vi "CRYO_MASTER_temp.vi"() -> ()   [LabVIEW 2017] (continued)
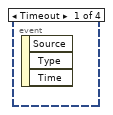
[diagram p2: hidden frame]
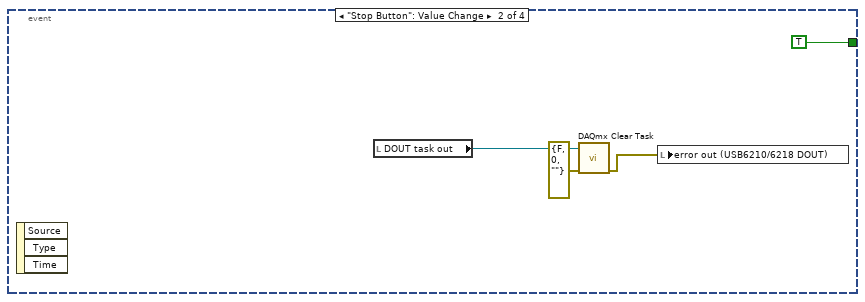
[diagram p3: hidden frame]
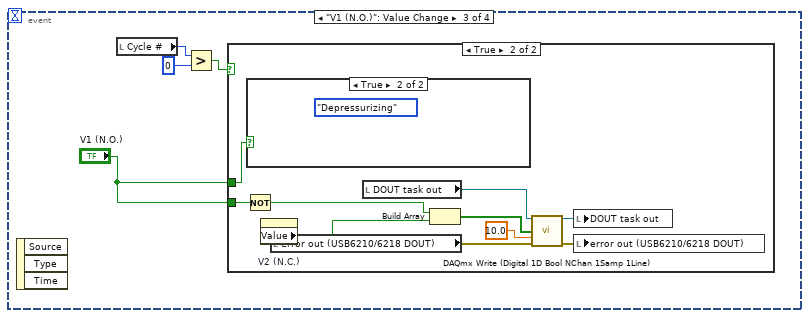
[diagram p4: hidden frame]
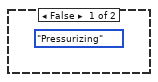
[diagram p6: hidden frame]
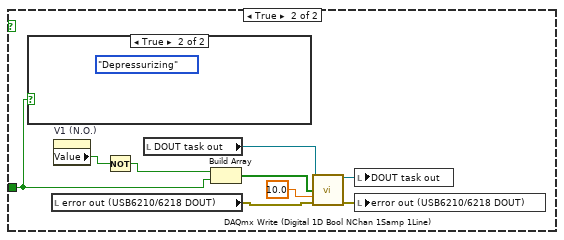
[diagram p7: hidden frame]
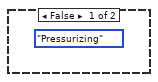
[diagram p8: hidden frame]
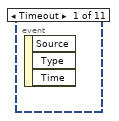
[diagram p9: hidden frame]
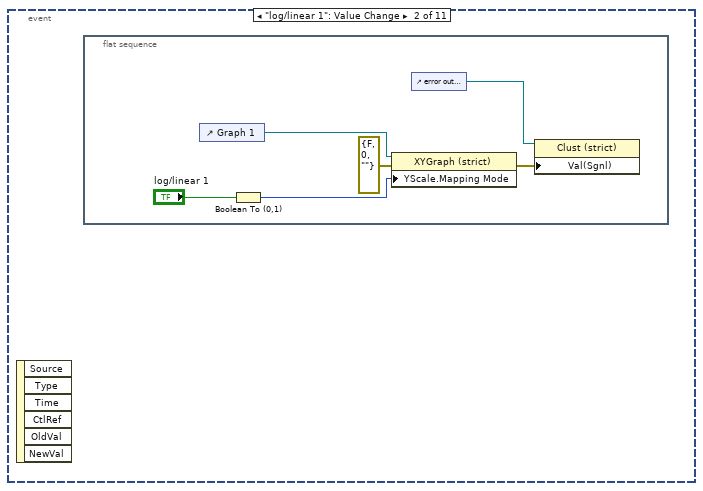
[diagram p10: hidden frame]
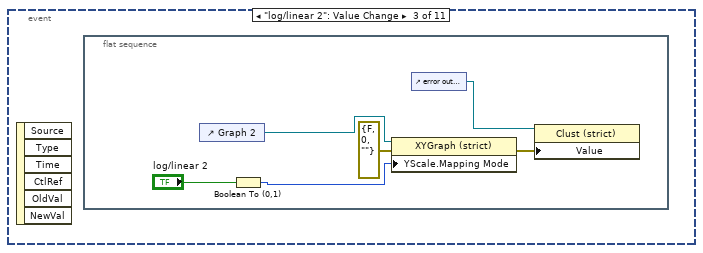
[diagram p11: hidden frame]
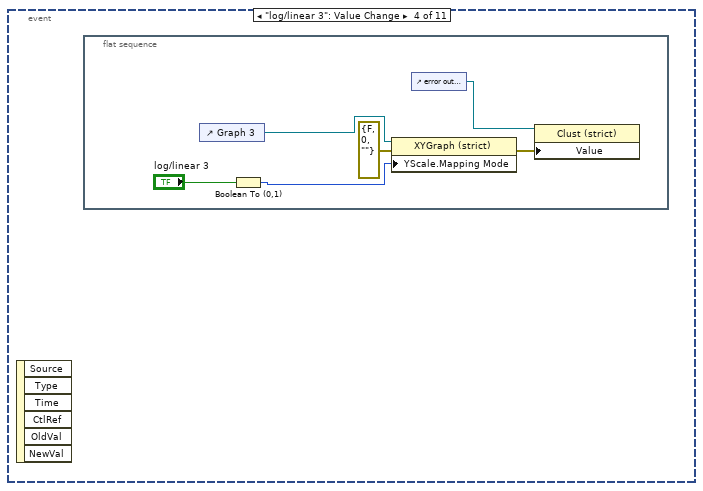
[diagram p12: hidden frame]
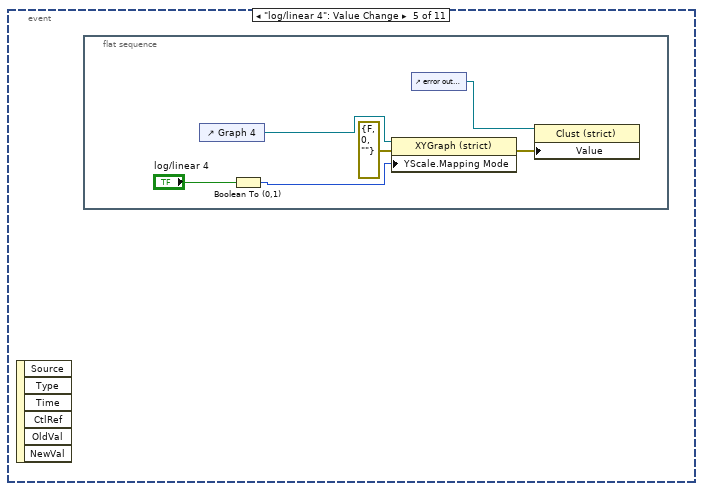
[diagram p13: hidden frame]
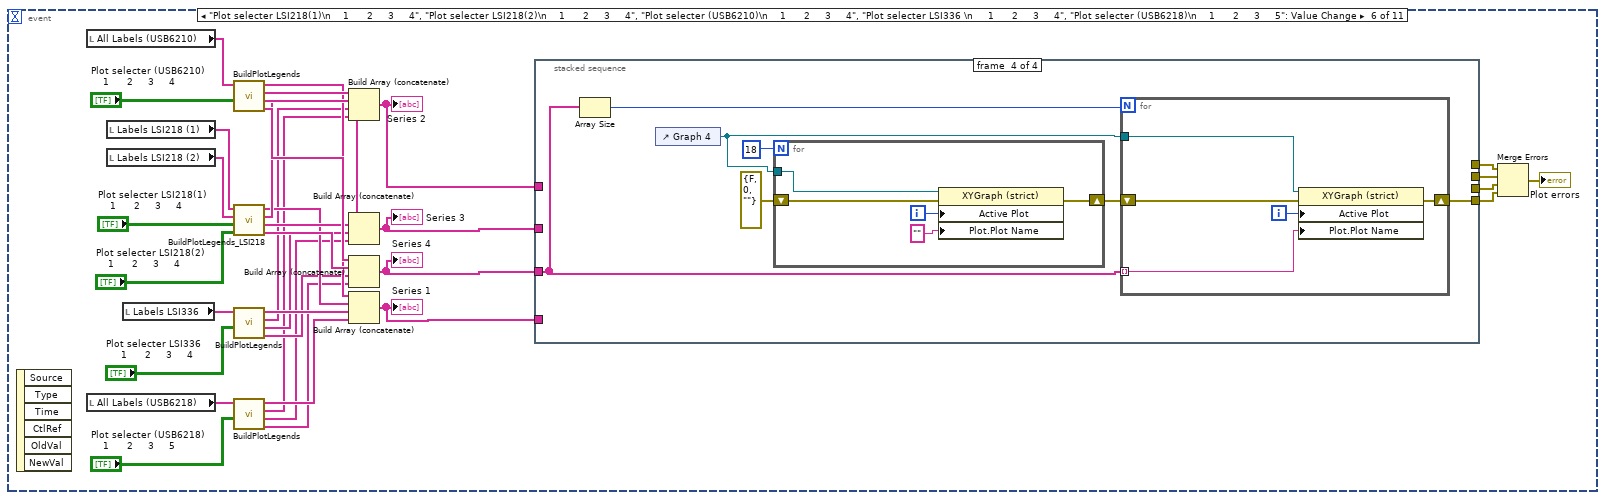
[diagram p14: hidden frame]
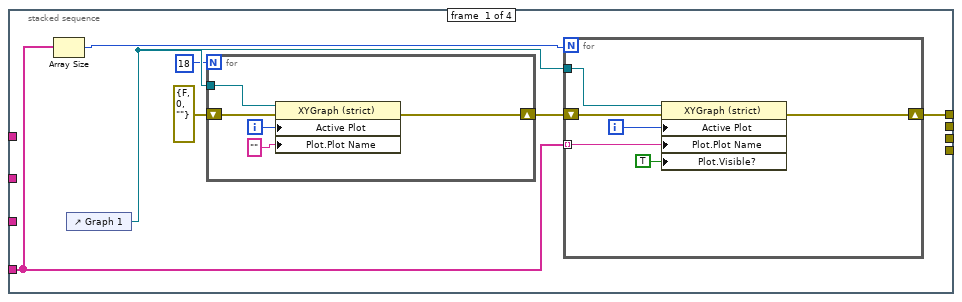
[diagram p15: hidden frame]
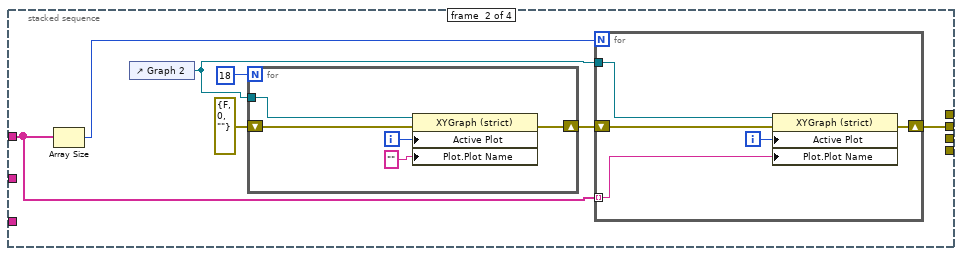
[diagram p16: hidden frame]
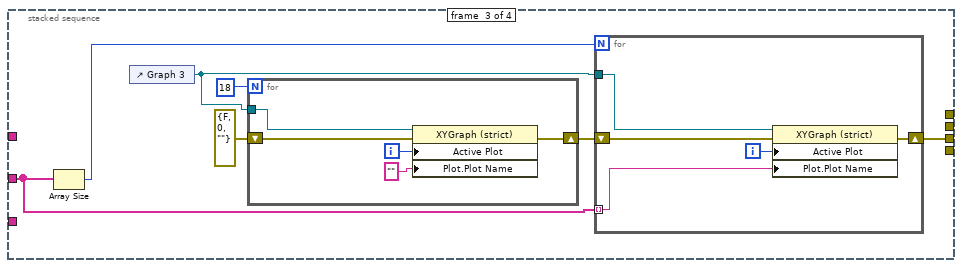
[diagram p17: hidden frame]
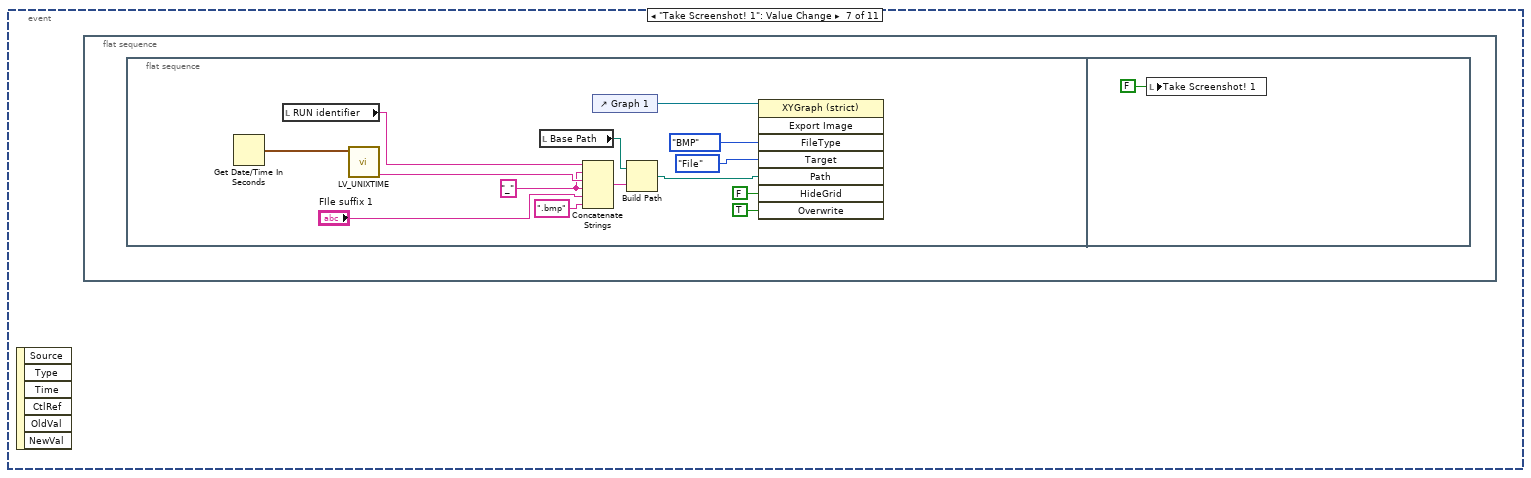
[diagram p18: hidden frame]
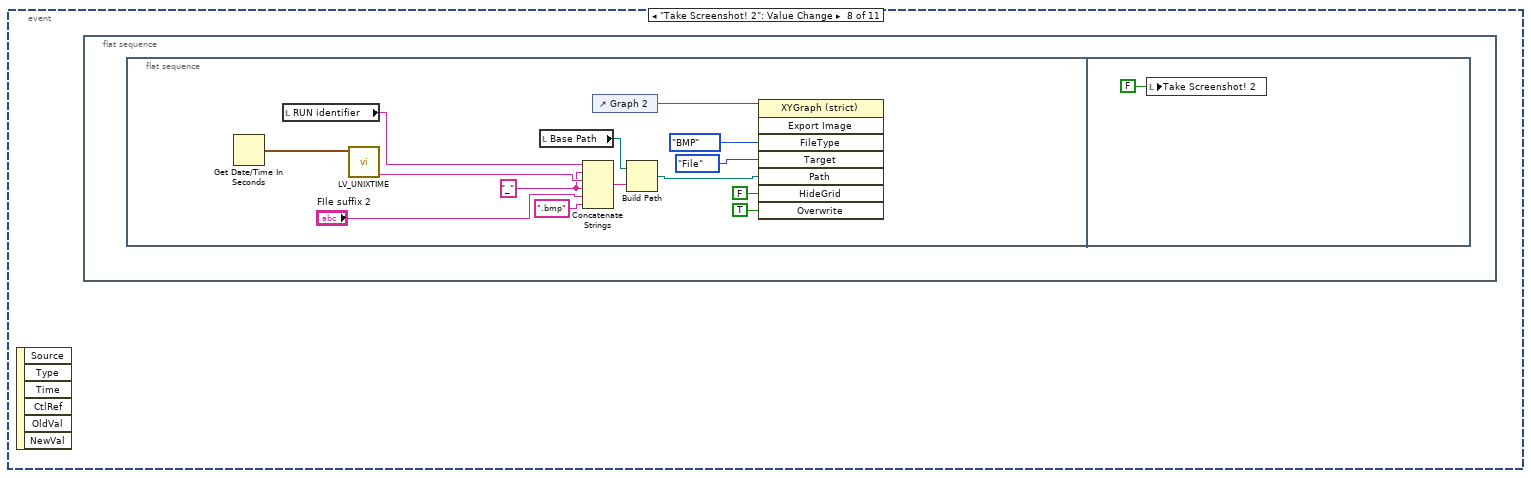
[diagram p19: hidden frame]
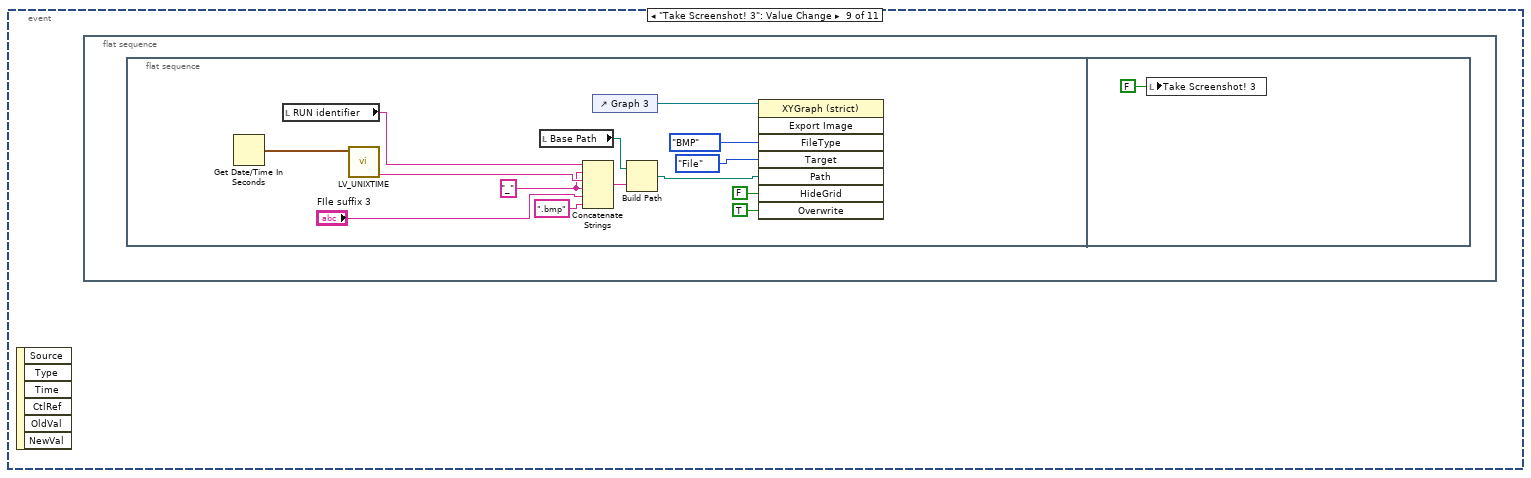
[diagram p20: hidden frame]
      }
    }
    "LSI336 Status" <- w289
    "error out (LSI336)" <- w279
    n190 = case shown="False" w264 {
      tunnel: [w502 w530] -> w252
      tunnel: [w499 w529] -> w259
      tunnel: [w500 w528] -> w253
      tunnel: [w490 w523] -> w258
      tunnel: [w489 w520] -> _
      tunnel: w265 -> [w488 w518]
      tunnel: w263 -> [_ w517]
      tunnel: w262 -> [_ w516]
      tunnel: w261 -> [w487 w515]
      tunnel: w260 -> [w486 _]
      frame False {
        n191 = call-dynamic "USBData_measure.vi"("USBData in"=w488, "DAQ sample #"=i64 5, "DAQ timeout"=100.0 ("DAQ timeout (def: 100)"), "MeasurementIndex"=w486, "error in (no error)"=w487) -> ("USBData out"=w508:refnum<class "USBData.lvclass">, "TimeMeasuremeent"=w505:timestamp, "Status"=→"USB6218 Status":T5, "LastDataAcquired"=w492:dbl[], "error out"=w504:errorcluster)  [unwired: 4 in, 2 out]
        "Time of Last Measurement (USB6218)" <- w505
        "Last Vol \n(USB6218)" <- w492
        n192 = call-dynamic "USBData_convert.vi"("Save every ... measurements"="Record interval (USB6218)", "MeasurementIndex"=w486, "error in (no error)"=w504, "LastDataAcquired"=w492, "TimeMeasuremeent"=w505, "USBData in"=w508) -> ("error out"=w503:errorcluster, "LeakDet_FULL"=w498:dbl, "LastDataConverted"=w493:dbl[], "USBData out"=w501:refnum<class "USBData.lvclass">)  [unwired: 2 in]
        n193 = call "USBData_read.vi"("USBData in"=w501, "error in (no error)"=w503) -> ("Status"=w494:T5, "USBData out"=w500:refnum<class "USBData.lvclass">, "Data"=w499:T13, "Basic"=w490:T14, "error out"=w502:errorcluster)  [unwired: 2 in, 2 out]
        n194 = local write "USB6218 Status"(w494) -> ()
        n195 = Unbundle By Name(w490) -> ("ReadLeakDet?"=w497:bool)
        n196 = Unbundle By Name(w490) -> ("Labels"=w489:string[])
        n197 = case shown="True" w497 {
          tunnel: w493 -> [w509 w512]
          tunnel: w498 -> [_ w511]
          tunnel: [w509 w510] -> w496
          frame False {
          }
          frame True {
            n198 = Build Array (concatenate)(w512, w511) -> (w510:dbl[])
          }
        }
        "Last Data \n(USB6218)" <- w496
      }
      frame True {
        n199 = Get Date/Time In Seconds() -> (seconds since 1Jan1904=w522:timestamp)
        n200 = call-dynamic "USBData_initialize.vi"("USBData in"=w518, "SeriesSetting"="USB6218 Config", "BasePath"=w517, "RunName"=w516, "FileName"="InstName (USB6218)", "error in (no error)"=w515, "RUN start time"=w522) -> ("Status"=w513:T5, "USBData out"=w531:refnum<class "USBData.lvclass">, "error out"=w532:errorcluster)  [unwired: 4 in, 2 out]
        n201 = local write "USB6218 Status"(w513) -> ()
        n202 = call "USBData_read.vi"("USBData in"=w531, "error in (no error)"=w532) -> ("Status"=w521:T5, "USBData out"=w528:refnum<class "USBData.lvclass">, "Data"=w529:T13, "Basic"=w523:T14, "error out"=w530:errorcluster)  [unwired: 2 in, 2 out]
        n203 = local write "USB6218 Status"(w521) -> ()
        n204 = Unbundle By Name(w523) -> ("ReadLeakDet?"=w527:bool, "Labels"=w520:string[])
        n205 = Array Size(array=w520) -> (size(s)=w526:i32)
        n206 = case shown="True" w527 {
          tunnel: w526 -> [w533 w535]
          tunnel: [w533 w534] -> w524
          frame False {
          }
          frame True {
            n207 = Add(x=w535, y=1) -> (x+y=w534:i32)
          }
        }
        n208 = Initialize Array(TRUE ("Activate 2"), w524) -> ()  [unwired: 1 out]
      }
    }
    "error out (USB6218)" <- w252
    n209 = case shown="False" w264 {
      tunnel: [w838 w853] -> w294
      tunnel: [w833 w852] -> w313
      tunnel: [w836 w851] -> w295
      tunnel: w260 -> [w837 _]
      tunnel: w312 -> [w827 w846]
      tunnel: w311 -> [w828 w845]
      tunnel: w262 -> [_ w844]
      tunnel: w263 -> [_ w843]
      tunnel: [w825 timestamp[] [] ("TimeArray")] -> w310
      tunnel: [w824 dbl[][] [] ("DataArray")] -> w309
      frame False {
        w831 = 24 ("index")
        n210 = call-dynamic "LSI218Data_measure.vi"("LSI218Data in"=w828, "MeasurementIndex"=w837, "error in (no error)"=w827, "save every ... measurements"="Record interval (LSI218)") -> ("TimeMeasuremeent"=→"Time of Last Measurement (LSI218)":timestamp, "Active?"=w832:bool[], "LSI218Data out"=w836:refnum<class "LSI218Data.lvclass">, "LastMeasurementConfig"=→"LastMeasurementConfig (218)":T10, "LastData"=w826:dbl[], "Status"=w833:u16, "TimeArray"=w825:timestamp[], "DataArray"=w824:dbl[][], "error out"=w838:errorcluster)  [unwired: 3 in]
        n211 = Split 1D Array(array=w832, index=w831) -> (first subarray=→"Active?\n (1)":bool[], second subarray=→"Active?\n(2)":bool[])
        n212 = Split 1D Array(array=w826, index=w831) -> (first subarray=→"Last Data \nLSI218 (1)":dbl[], second subarray=→"Last Data \nLSI218 (2)":dbl[])
      }
      frame True {
        n213 = Get Date/Time In Seconds() -> (seconds since 1Jan1904=w854:timestamp)
        n214 = call-dynamic "LSI218Data_initialize.vi"("LSI218Settings(A-F)"="LSI218Settings(A-F)", "FileFormat"="FileFormat (218)", "RUN start time"=w854, "base path"=w843, "error in (no error)"=w846, "InstName"="InstName (LSI218)", "RunName"=w844, "LSI218Data in"=w845) -> ("error out"=w853:errorcluster, "Status"=w852:T6, "AllLabels"=w842:string[], "LSI218Data out"=w851:refnum<class "LSI218Data.lvclass">)
        n215 = Split 1D Array(array=w842, index=24) -> (first subarray=→"Labels LSI218 (1)":string[], second subarray=→"Labels LSI218 (2)":string[])
      }
    }
    "LSI218 Status" <- w313
    "error out (LSI218)" <- w294
    n216 = property on="Property Node" class="Arr (strict)"(reference=w272, "Number of Rows"=u32 8) -> ()  [unwired: 1 in, 2 out]
    n217 = Multiply(x="Measurement Interval (s)", y=u32 1000) -> (x*y=w315:dbl)
    n218 = Wait (ms)(milliseconds to wait=w315) -> ()  [unwired: 1 out]
    n219 = case shown="True" "Digital Out ON?" {
      tunnel: w264 -> [_ w542]
      tunnel: w269 -> [_ w541]
      tunnel: w268 -> [w537 w540]
      tunnel: [w537 w539] -> w267
      tunnel: w266 -> [_ w538]
      frame False {
      }
      frame True {
        n220 = case shown="False" w542 {
          tunnel: w541 -> [_ w665]
          tunnel: w540 -> [w552 w647]
          tunnel: [w552 w637] -> w539
          tunnel: w538 -> [w553 _]
          frame False {
            n221 = Multiply(x="N for sampling", y=i64 2) -> (x*y=w547:i64)
            n222 = local read "Cycle #"() -> (w551:u32)
            n223 = Add(x=w547, y="Mov. Avg Interval") -> (x+y=w549:i64)
            n224 = Greater?(x=w551, y=w549) -> (0:w545:bool)
            n225 = And(x=w545, y="Auto ON?") -> (x .and. y?=w543:bool)
            n226 = case shown="True" w543 {
              tunnel: w553 -> [_ w575]
              tunnel: "Mov. Avg Interval" -> [_ w557]
              tunnel: w547 -> [_ w559]
              tunnel: "N for sampling" -> [_ w554]
              frame False {
              }
              frame True {
                # "Need to record the valve status"
                n227 = Reciprocal(x=w557) -> (1/x=w572:dbl)
                n228 = local read "Pstd"() -> (→"Pstd history":dbl)
                n229 = local read "Pav"() -> (→"Pav history":dbl)
                n230 = Unbundle By Name(w575) -> ("TimeArray"=w573:timestamp[], "DataArrayConv"=w574:dbl[][])
                n231 = local read "Target Index"() -> (w576:i32)
                n232 = Index Array(array=w574, index (col)=w576) -> (element=w567:dbl[])  [unwired: 1 in]
                n233 = Initialize Array(w572, w557) -> (w571:dbl[])
                n234 = Delete From Array(array=w567, length=w559) -> (deleted portion=w566:dbl[])  [unwired: 1 in, 1 out]
                n235 = call-poly <vilib>:"FIR Filter.vi"("FIR Coefficients"=w571, "X"=w567) -> ("Filtered X"=w564:dbl[])  [unwired: 2 in, 1 out]
                n236 = Delete From Array(array=w573, length=w559) -> (deleted portion=w570:timestamp[])  [unwired: 1 in, 1 out]
                n237 = Delete From Array(array=w564, length=w559) -> (deleted portion=w568:dbl[])  [unwired: 1 in, 1 out]
                n238 = Delete From Array(array=w564, length=w554) -> (deleted portion=w562:dbl[])  [unwired: 1 in, 1 out]
                "Last N M.A. Pressures" <- w562
                n239 = Bundle("TimeArray"=w570, "DataArrayConv"=w566) -> (w565:T15)  [unwired: 1 in]
                n240 = Bundle("TimeArray"=w570, "Filtered X"=w568) -> (w569:T16)  [unwired: 1 in]
                n241 = Array Size(array=w562) -> (size(s)=w561:i32)
                n242 = Equal?(x=w561, y=w554) -> (x = y?=w560:bool)
                n243 = Build Array(w565, w569) -> (→"Graph 5":T9)
                n244 = case shown="True" w560 {
                  tunnel: [nan ("mean") w579] -> w558
                  tunnel: w562 -> [_ w580]
                  frame False {
                  }
                  frame True {
                    n245 = call <vilib>:"Std Deviation and Variance.vi"("X"=w580) -> ("mean"=w579:dbl, "standard deviation"=w578:dbl)  [unwired: 1 in, 1 out]
                    n246 = local write "Pav"(w579) -> ()
                    n247 = local write "Pstd"(w578) -> ()
                  }
                }
                n248 = stacked-sequence {
                  tunnel: w558 -> [w583 w595 w607 w619 w632]
                  frame #0 {
                    n249 = local read "P_1_th_high (Pa)"() -> (w590:dbl)
                    n250 = local read "P_1_tol (Pa)"() -> (w591:dbl)
                    n251 = local write "Status V1 CTRL"(enum16{"Pressurize", "Depressurize"}."Depressurize" ("Status V1 CTRL")) -> ()
                    n252 = local read "V1 (N.O.)"() -> (w588:bool)
                    n253 = Add(x=w590, y=w591) -> (x+y=w582:dbl)
                    n254 = Greater?(x=w583, y=w582) -> (0:w589:bool)
                    n255 = Equal?(x=w588, y=FALSE) -> (x = y?=w586:bool)
                    n256 = Subtract(x=w583, y=w582) -> (x-y=→"Pav - (P_1_th_high+P_1_tol)=":dbl)
                    n257 = And(x=w589, y=w586) -> (x .and. y?=w585:bool)
                    n258 = case shown="True" w585 {
                      frame False {
                      }
                      frame True {
                        n259 = property on="V1 (N.O.)" class="Bool (strict)"("Val(Sgnl)"=TRUE ("V1 (N.O.)")) -> ()  [unwired: 2 in, 2 out]
                      }
                    }
                  }
                  frame #1 {
                    n260 = local read "P_2_th_high (Pa)"() -> (w602:dbl)
                    n261 = local read "P_2_tol (Pa)"() -> (w603:dbl)
                    n262 = local write "Status V2 CTRL"(enum16{"Pressurize", "Depressurize"}."Depressurize" ("Status V2 CTRL")) -> ()
                    n263 = local read "V2 (N.C.)"() -> (w600:bool)
                    n264 = Add(x=w602, y=w603) -> (x+y=w594:dbl)
                    n265 = Greater?(x=w595, y=w594) -> (0:w601:bool)
                    n266 = Equal?(x=w600, y=TRUE) -> (x = y?=w598:bool)
                    n267 = Subtract(x=w595, y=w594) -> (x-y=→"Pav - (P_2_th_high+P_2_tol)=":dbl)
                    n268 = And(x=w601, y=w598) -> (x .and. y?=w597:bool)
                    n269 = case shown="True" w597 {
                      frame False {
                      }
                      frame True {
                        n270 = property on="V2 (N.C.)" class="Bool (strict)"("Val(Sgnl)"=FALSE ("V1 (N.O.)")) -> ()  [unwired: 2 in, 2 out]
                      }
                    }
                  }
                  frame #2 {
                    n271 = local read "P_1_th_low (Pa)"() -> (w614:dbl)
                    n272 = local read "P_1_tol (Pa)"() -> (w615:dbl)
                    n273 = local write "Status V1 CTRL"(enum16{"Pressurize", "Depressurize"}."Pressurize" ("Status V1 CTRL")) -> ()
                    n274 = local read "V1 (N.O.)"() -> (w612:bool)
                    n275 = Subtract(x=w614, y=w615) -> (x-y=w606:dbl)
                    n276 = Less?(x=w607, y=w606) -> (x < y?=w613:bool)
                    n277 = Subtract(x=w607, y=w606) -> (x-y=→"Pav - (P_1_th_low_-P_1_tol)=":dbl)
                    n278 = Equal?(x=w612, y=TRUE) -> (x = y?=w610:bool)
                    n279 = And(x=w613, y=w610) -> (x .and. y?=w609:bool)
                    n280 = case shown="True" w609 {
                      frame False {
                      }
                      frame True {
                        n281 = property on="V1 (N.O.)" class="Bool (strict)"("Val(Sgnl)"=FALSE ("V1 (N.O.)")) -> ()  [unwired: 2 in, 2 out]
                      }
                    }
                  }
                  frame #3 {
                    n282 = local read "P_2_th_low (Pa)"() -> (w626:dbl)
                    n283 = local write "Status V2 CTRL"(enum16{"Pressurize", "Depressurize"}."Pressurize" ("Status V2 CTRL")) -> ()
                    n284 = local read "P_2_tol (Pa)"() -> (w627:dbl)
                    n285 = local read "V2 (N.C.)"() -> (w624:bool)
                    n286 = Subtract(x=w626, y=w627) -> (x-y=w618:dbl)
                    n287 = Less?(x=w619, y=w618) -> (x < y?=w625:bool)
                    n288 = Equal?(x=w624, y=FALSE) -> (x = y?=w622:bool)
                    n289 = Subtract(x=w619, y=w618) -> (x-y=→"Pav - (P_2_th_low_-P_2_tol)=":dbl)
                    n290 = And(x=w625, y=w622) -> (x .and. y?=w621:bool)
                    n291 = case shown="True" w621 {
                      frame False {
                      }
                      frame True {
                        n292 = property on="V2 (N.C.)" class="Bool (strict)"("Val(Sgnl)"=TRUE ("V1 (N.O.)")) -> ()  [unwired: 2 in, 2 out]
                      }
                    }
                  }
                  frame #4 {
                    n293 = Less?(x=w632, y="P_safelimit_low (Pa)") -> (x < y?=w630:bool)
                    n294 = Greater?(x=w632, y="P_safelimit_up (Pa)") -> (0:w633:bool)
                    n295 = Or(x=w633, y=w630) -> (x .or. y?=w629:bool)
                    n296 = case shown="True" w629 {
                      frame False {
                      }
                      frame True {
                        n297 = property on="V1 (N.O.)" class="Bool (strict)"("Val(Sgnl)"=TRUE ("V1 (N.O.)")) -> ()  [unwired: 2 in, 2 out]
                        n298 = property on="V2 (N.C.)" class="Bool (strict)"("Val(Sgnl)"=FALSE ("V1 (N.O.)")) -> ()  [unwired: 2 in, 2 out]
                      }
                    }
                  }
                }
              }
            }
          }
          frame True {
            w652 = 1 items=["one channel for each line", "one channel for all lines"] ("line grouping")
            w651 = 1 items=["one channel for each line", "one channel for all lines"] ("line grouping")
            n299 = Get Date/Time In Seconds() -> (seconds since 1Jan1904=w658:timestamp)
            n300 = local write "V2 (N.C.)"(FALSE ("V1 (N.O.)")) -> ()
            n301 = local write "V1 (N.O.)"(TRUE ("V1 (N.O.)")) -> ()
            n302 = call "LV_UNIXTIME.vi"("current time"=w658) -> ("date/time string"=w659:string)  [unwired: 9 in, 1 out]
            n303 = Search 1D Array(1D array=w665, element="TargetSignal Label") -> (index of element=→"Target Index":i32)  [unwired: 1 in]
            n304 = Concatenate Strings(w659, "_DO" ("new task name")) -> (w655:string)
            n305 = call <vilib>:"DAQmx Create Task.vi"("new task name"=w655, "auto cleanup"=FALSE, "error in"=w647) -> ("task out"=w656:refnum<k21>, "error out"=w657:errorcluster)  [unwired: 11 in]
            n306 = call-poly <vilib>:"DAQmx Create Virtual Channel.vi"("task in"=w656, "lines"="DOUT for Vavle V1 (N.O.)", "line grouping"=w652, "error in"=w657) -> ("task out"=w660:refnum<k21>, "error out"=w661:errorcluster)  [unwired: 10 in]
            n307 = call-poly <vilib>:"DAQmx Create Virtual Channel.vi"("task in"=w660, "lines"="DOUT for Vavle V2 (N.C.)", "line grouping"=w651, "error in"=w661) -> ("task out"=w663:refnum<k21>, "error out"=w662:errorcluster)  [unwired: 10 in]
            n308 = call <vilib>:"DAQmx Start Task.vi"("task/channels in"=w663, "error in"=w662) -> ("task out"=w640:refnum<k21>, "error out"=w638:errorcluster)  [unwired: 12 in]
            n309 = Build Array(FALSE ("auto cleanup"), FALSE ("auto cleanup")) -> (w641:bool[])
            n310 = call <vilib>:"DAQmx Write (Digital 1D Bool NChan 1Samp 1Line).vi"("task/channels in"=w640, "data"=w641, "timeout"=10.0, "error in"=w638) -> ("task out"=→"DOUT task out":refnum<k21>, "error out"=w637:errorcluster)  [unwired: 9 in, 1 out]
          }
        }
      }
    }
    "error out (USB6210/6218 DOUT)" <- w267
    n311 = flat-sequence {
      tunnel: w319 -> [w420]
      tunnel: [w414] -> w306
      tunnel: [w412] -> w304
      tunnel: [w411] -> w301
      tunnel: [w410] -> w298
      tunnel: w266 -> [w405]
      frame #0 {
        w413 = T12 [] ("appended array")
        n312 = Unbundle By Name(w405) -> ("TimeArray"=w423:timestamp[], "DataArrayConv"=w418:dbl[][], "LDArray"=w417:dbl[])
        n313 = Unbundle By Name(w420) -> ("ReadLeakDet?"=w419:bool, "LabelLD"=w422:string, "Labels"=w415:string[])  [unwired: 1 out]
        n314 = case shown="True" w419 {
          tunnel: w422 -> [_ w431]
          tunnel: w418 -> [w425 w430]
          tunnel: w417 -> [_ w429]
          tunnel: [w425 w428] -> w416
          tunnel: w415 -> [w424 w427]
          tunnel: [w424 w426] -> w407
          frame False {
          }
          frame True {
            n315 = Build Array (concatenate)(w430, w429) -> (w428:dbl[][])
            n316 = Build Array (concatenate)(w427, w431) -> (w426:string[])
          }
        }
        "All Labels (USB6210)" <- w407
        "DataArrayConv (USB)" <- w416
        n317 = local read "Plot selecter (USB6210)\n    1      2     3     4"() -> (w409:bool[][])
        n318 = control-ref of="Plot selecter (USB6210)\n    1      2     3     4"() -> (w406:refnum<vi>)
        n319 = Array Size(array=w407) -> (size(s)=w421:i32)
        n320 = Array Size(array=w407) -> (size(s)=w408:i32)
        n321 = property on="Property Node" class="Arr (strict)"(reference=w406, "Number of Rows"=w408) -> ()  [unwired: 1 in, 2 out]
        n322 = for {
          N: w421 -> [_]
          tunnel: w416 -> [w452]
          tunnel: w423 -> [w453]
          shift-right: [w447] -> w412
          shift-left: w413 -> [w450]
          shift-right: [w445] -> w410
          shift-left: w413 -> [w448]
          shift-right: [w446] -> w414
          shift-left: w413 -> [w444]
          shift-right: [w443] -> w411
          shift-left: w413 -> [w442]
          tunnel: w409 -> [w441]
          i -> [w436]
          n323 = Index Array(array=w452, index (col)=w436) -> (element=w451:dbl[])  [unwired: 1 in]
          n324 = Index Array(array=w441, index (row) #1=w436, index (col) #1=0 ("index (row)"), index (row) #2=w436, index (col) #2=1 ("index (row)"), index (row) #3=w436, index (col) #3=2 ("index (row)"), index (row) #4=w436, index (col) #4=3 ("index (row)")) -> (element #1=w435:bool, element #2=w434:bool, element #3=w433:bool, element #4=w432:bool)
          n325 = Bundle("TimeArray"=w453, "DataArrayConv"=w451) -> (w449:T15)  [unwired: 1 in]
          n326 = stacked-sequence {
            tunnel: w435 -> [w457 _ _ _]
            tunnel: w450 -> [_ w465 _ _]
            tunnel: w433 -> [_ _ w473 _]
            tunnel: w449 -> [w454 w463 w472 w478]
            tunnel: w432 -> [_ _ _ w481]
            tunnel: w448 -> [_ _ _ w480]
            tunnel: [_ _ _ w479] -> w445
            tunnel: [_ w464 _ _] -> w447
            tunnel: [w456 _ _ _] -> w446
            tunnel: w444 -> [w455 _ _ _]
            tunnel: [_ _ w471 _] -> w443
            tunnel: w442 -> [_ _ w470 _]
            tunnel: w434 -> [_ w462 _ _]
            frame #0 {
              n327 = case shown="True" w457 {
                tunnel: [w458 w461] -> w456
                tunnel: w454 -> [_ w460]
                tunnel: w455 -> [w458 w459]
                frame False {
                }
                frame True {
                  n328 = Build Array (concatenate)(w459, w460) -> (w461:T12)
                }
              }
            }
            frame #1 {
              n329 = case shown="True" w462 {
                tunnel: w465 -> [w466 w469]
                tunnel: [w466 w468] -> w464
                tunnel: w463 -> [_ w467]
                frame False {
                }
                frame True {
                  n330 = Build Array (concatenate)(w469, w467) -> (w468:T12)
                }
              }
            }
            frame #2 {
              n331 = case shown="True" w473 {
                tunnel: [w474 w477] -> w471
                tunnel: w472 -> [_ w476]
                tunnel: w470 -> [w474 w475]
                frame False {
                }
                frame True {
                  n332 = Build Array (concatenate)(w475, w476) -> (w477:T12)
                }
              }
            }
            frame #3 {
              n333 = case shown="True" w481 {
                tunnel: [w482 w485] -> w479
                tunnel: w478 -> [_ w484]
                tunnel: w480 -> [w482 w483]
                frame False {
                }
                frame True {
                  n334 = Build Array (concatenate)(w483, w484) -> (w485:T12)
                }
              }
            }
          }
        }
      }
    }
    n335 = flat-sequence {
      tunnel: w258 -> [w339]
      tunnel: [w333] -> w257
      tunnel: [w331] -> w256
      tunnel: [w330] -> w255
      tunnel: [w329] -> w254
      tunnel: w259 -> [w325]
      frame #0 {
        w332 = T12 [] ("appended array")
        n336 = Unbundle By Name(w325) -> ("TimeArray"=w342:timestamp[], "DataArrayConv"=w337:dbl[][], "LDArray"=w336:dbl[])
        n337 = Unbundle By Name(w339) -> ("ReadLeakDet?"=w338:bool, "LabelLD"=w341:string, "Labels"=w334:string[])  [unwired: 1 out]
        n338 = case shown="True" w338 {
          tunnel: w341 -> [_ w350]
          tunnel: w337 -> [w344 w349]
          tunnel: w336 -> [_ w348]
          tunnel: [w344 w347] -> w335
          tunnel: w334 -> [w343 w346]
          tunnel: [w343 w345] -> w326
          frame False {
          }
          frame True {
            n339 = Build Array (concatenate)(w349, w348) -> (w347:dbl[][])
            n340 = Build Array (concatenate)(w346, w350) -> (w345:string[])
          }
        }
        "All Labels (USB6218)" <- w326
        "DataArrayConv (USB) 2" <- w335
        n341 = control-ref of="Plot selecter (USB6218)\n    1      2     3     5"() -> (w324:refnum<vi>)
        n342 = local read "Plot selecter (USB6218)\n    1      2     3     5"() -> (w328:bool[][])
        n343 = Array Size(array=w326) -> (size(s)=w340:i32)
        n344 = Array Size(array=w326) -> (size(s)=w327:i32)
        n345 = property on="Property Node" class="Arr (strict)"(reference=w324, "Number of Rows"=w327) -> ()  [unwired: 1 in, 2 out]
        n346 = for {
          N: w340 -> [_]
          tunnel: w335 -> [w371]
          tunnel: w342 -> [w372]
          shift-right: [w366] -> w331
          shift-left: w332 -> [w369]
          shift-right: [w364] -> w329
          shift-left: w332 -> [w367]
          shift-right: [w365] -> w333
          shift-left: w332 -> [w363]
          shift-right: [w362] -> w330
          shift-left: w332 -> [w361]
          tunnel: w328 -> [w360]
          i -> [w355]
          n347 = Index Array(array=w371, index (col)=w355) -> (element=w370:dbl[])  [unwired: 1 in]
          n348 = Index Array(array=w360, index (row) #1=w355, index (col) #1=0 ("index (row)"), index (row) #2=w355, index (col) #2=1 ("index (row)"), index (row) #3=w355, index (col) #3=2 ("index (row)"), index (row) #4=w355, index (col) #4=3 ("index (row)")) -> (element #1=w354:bool, element #2=w353:bool, element #3=w352:bool, element #4=w351:bool)
          n349 = Bundle("TimeArray"=w372, "DataArrayConv"=w370) -> (w368:T15)  [unwired: 1 in]
          n350 = stacked-sequence {
            tunnel: w354 -> [w376 _ _ _]
            tunnel: w369 -> [_ w384 _ _]
            tunnel: w352 -> [_ _ w392 _]
            tunnel: w368 -> [w373 w382 w391 w397]
            tunnel: w351 -> [_ _ _ w400]
            tunnel: w367 -> [_ _ _ w399]
            tunnel: [_ _ _ w398] -> w364
            tunnel: [_ w383 _ _] -> w366
            tunnel: [w375 _ _ _] -> w365
            tunnel: w363 -> [w374 _ _ _]
            tunnel: [_ _ w390 _] -> w362
            tunnel: w361 -> [_ _ w389 _]
            tunnel: w353 -> [_ w381 _ _]
            frame #0 {
              n351 = case shown="True" w376 {
                tunnel: [w377 w380] -> w375
                tunnel: w373 -> [_ w379]
                tunnel: w374 -> [w377 w378]
                frame False {
                }
                frame True {
                  n352 = Build Array (concatenate)(w378, w379) -> (w380:T12)
                }
              }
            }
            frame #1 {
              n353 = case shown="True" w381 {
                tunnel: w384 -> [w385 w388]
                tunnel: [w385 w387] -> w383
                tunnel: w382 -> [_ w386]
                frame False {
                }
                frame True {
                  n354 = Build Array (concatenate)(w388, w386) -> (w387:T12)
                }
              }
            }
            frame #2 {
              n355 = case shown="True" w392 {
                tunnel: [w393 w396] -> w390
                tunnel: w391 -> [_ w395]
                tunnel: w389 -> [w393 w394]
                frame False {
                }
                frame True {
                  n356 = Build Array (concatenate)(w394, w395) -> (w396:T12)
                }
              }
            }
            frame #3 {
              n357 = case shown="True" w400 {
                tunnel: [w401 w404] -> w398
                tunnel: w397 -> [_ w403]
                tunnel: w399 -> [w401 w402]
                frame False {
                }
                frame True {
                  n358 = Build Array (concatenate)(w402, w403) -> (w404:T12)
                }
              }
            }
          }
        }
      }
    }
    n359 = local read "Plot selecter LSI218(1)\n    1      2     3     4"() -> (w293:bool[][])
    n360 = local read "Plot selecter LSI218(2)\n    1      2     3     4"() -> (w292:bool[][])
    n361 = for {
      N: 48 -> [_]
      tunnel: w310 -> [w766]
      tunnel: w309 -> [w763]
      tunnel: w293 -> [w747]
      tunnel: w292 -> [w748]
      shift-right: [w764] -> w308
      shift-left: w305 -> [w765]
      shift-right: [w759] -> w302
      shift-left: w305 -> [w760]
      shift-right: [w758] -> w299
      shift-left: w305 -> [w757]
      shift-right: [w756] -> w297
      shift-left: w305 -> [w755]
      i -> [w753]
      n362 = Index Array(array=w763, index (col)=w753) -> (element=w762:dbl[])  [unwired: 1 in]
      n363 = Less?(x=w753, y=24) -> (x < y?=w754:bool)
      n364 = case shown="True" w754 {
        tunnel: [w771 w789] -> w752
        tunnel: [w770 w788] -> w751
        tunnel: [w769 w786] -> w750
        tunnel: [w768 w785] -> w749
        tunnel: w747 -> [_ w784]
        tunnel: w748 -> [w778 _]
        tunnel: w753 -> [w773 w781]
        frame False {
          n365 = Subtract(x=w773, y=24) -> (x-y=w777:i32)
          n366 = Index Array(array=w778, index (row) #1=w777, index (col) #1=0 ("index (row)"), index (row) #2=w777, index (col) #2=1 ("index (row)"), index (row) #3=w777, index (col) #3=2 ("index (row)"), index (row) #4=w777, index (col) #4=3 ("index (row)")) -> (element #1=w771:bool, element #2=w770:bool, element #3=w769:bool, element #4=w768:bool)
        }
        frame True {
          n367 = Index Array(array=w784, index (row) #1=w781, index (col) #1=0 ("index (row)"), index (row) #2=w781, index (col) #2=1 ("index (row)"), index (row) #3=w781, index (col) #3=2 ("index (row)"), index (row) #4=w781, index (col) #4=3 ("index (row)")) -> (element #1=w789:bool, element #2=w788:bool, element #3=w786:bool, element #4=w785:bool)
        }
      }
      n368 = Bundle("TimeArray"=w766, "DataArray"=w762) -> (w761:T17)  [unwired: 1 in]
      n369 = stacked-sequence {
        tunnel: w765 -> [w793 _ _ _]
        tunnel: [w792 _ _ _] -> w764
        tunnel: w761 -> [w791 w801 w809 w817]
        tunnel: w760 -> [_ w800 _ _]
        tunnel: [_ w799 _ _] -> w759
        tunnel: [_ _ w808 _] -> w758
        tunnel: w757 -> [_ _ w807 _]
        tunnel: [_ _ _ w816] -> w756
        tunnel: w755 -> [_ _ _ w815]
        tunnel: w752 -> [w790 _ _ _]
        tunnel: w751 -> [_ w798 _ _]
        tunnel: w750 -> [_ _ w806 _]
        tunnel: w749 -> [_ _ _ w814]
        frame #0 {
          n370 = case shown="False" w790 {
            tunnel: w791 -> [_ w795]
            tunnel: w793 -> [w794 w797]
            tunnel: [w794 w796] -> w792
            frame False {
            }
            frame True {
              n371 = Build Array (concatenate)(w797, w795) -> (w796:T8)
            }
          }
        }
        frame #1 {
          n372 = case shown="True" w798 {
            tunnel: [w802 w805] -> w799
            tunnel: w801 -> [_ w804]
            tunnel: w800 -> [w802 w803]
            frame False {
            }
            frame True {
              n373 = Build Array (concatenate)(w803, w804) -> (w805:T8)
            }
          }
        }
        frame #2 {
          n374 = case shown="True" w806 {
            tunnel: [w810 w813] -> w808
            tunnel: w809 -> [_ w812]
            tunnel: w807 -> [w810 w811]
            frame False {
            }
            frame True {
              n375 = Build Array (concatenate)(w811, w812) -> (w813:T8)
            }
          }
        }
        frame #3 {
          n376 = case shown="True" w814 {
            tunnel: [w818 w821] -> w816
            tunnel: w817 -> [_ w820]
            tunnel: w815 -> [w818 w819]
            frame False {
            }
            frame True {
              n377 = Build Array (concatenate)(w819, w820) -> (w821:T8)
            }
          }
        }
      }
    }
    n378 = local read "Plot selecter LSI336 \n     1      2     3     4"() -> (w288:bool[][])
    n379 = local read "Labels LSI336"() -> (w278:string[])
    n380 = Array Size(array=w278) -> (size(s)=w277:i32)
    n381 = for {
      N: w277 -> [_]
      tunnel: w288 -> [w678]
      shift-right: [w672] -> w284
      shift-left: w287 -> [w687]
      shift-right: [w668] -> w283
      shift-left: w287 -> [w685]
      shift-right: [w669] -> w282
      shift-left: w287 -> [w684]
      shift-right: [w667] -> w281
      shift-left: w287 -> [w683]
      tunnel: w286 -> [w675]
      tunnel: w285 -> [w673]
      i -> [w676]
      n382 = Index Array(array=w675, index (col)=w676) -> (element=w674:dbl[])  [unwired: 1 in]
      n383 = Index Array(array=w678, index (row) #1=w676, index (col) #1=0 ("index (row)"), index (row) #2=w676, index (col) #2=1 ("index (row)"), index (row) #3=w676, index (col) #3=2 ("index (row)"), index (row) #4=w676, index (col) #4=3 ("index (row)")) -> (element #1=w677:bool, element #2=w671:bool, element #3=w670:bool, element #4=w666:bool)
      n384 = Bundle("TimeArray"=w673, "DataArray"=w674) -> (w686:T17)  [unwired: 1 in]
      n385 = stacked-sequence {
        tunnel: w687 -> [w691 _ _ _]
        tunnel: [w690 _ _ _] -> w672
        tunnel: w686 -> [w689 w699 w707 w715]
        tunnel: w685 -> [_ w698 _ _]
        tunnel: [_ w697 _ _] -> w668
        tunnel: [_ _ w706 _] -> w669
        tunnel: w684 -> [_ _ w705 _]
        tunnel: [_ _ _ w714] -> w667
        tunnel: w683 -> [_ _ _ w713]
        tunnel: w677 -> [w688 _ _ _]
        tunnel: w671 -> [_ w696 _ _]
        tunnel: w670 -> [_ _ w704 _]
        tunnel: w666 -> [_ _ _ w712]
        frame #0 {
          n386 = case shown="False" w688 {
            tunnel: w689 -> [_ w693]
            tunnel: w691 -> [w692 w695]
            tunnel: [w692 w694] -> w690
            frame False {
            }
            frame True {
              n387 = Build Array (concatenate)(w695, w693) -> (w694:T8)
            }
          }
        }
        frame #1 {
          n388 = case shown="True" w696 {
            tunnel: [w700 w703] -> w697
            tunnel: w699 -> [_ w701]
            tunnel: w698 -> [w700 w702]
            frame False {
            }
            frame True {
              n389 = Build Array (concatenate)(w702, w701) -> (w703:T8)
            }
          }
        }
        frame #2 {
          n390 = case shown="False" w704 {
            tunnel: [w708 w711] -> w706
            tunnel: w707 -> [_ w709]
            tunnel: w705 -> [w708 w710]
            frame False {
            }
            frame True {
              n391 = Build Array (concatenate)(w710, w709) -> (w711:T8)
            }
          }
        }
        frame #3 {
          n392 = case shown="True" w712 {
            tunnel: [w716 w719] -> w714
            tunnel: w715 -> [_ w717]
            tunnel: w713 -> [w716 w718]
            frame False {
            }
            frame True {
              n393 = Build Array (concatenate)(w718, w717) -> (w719:T8)
            }
          }
        }
      }
    }
    n394 = Build Array (concatenate)(w306, w308, w284, w257) -> (→"Graph 1":T12)
    n395 = Build Array (concatenate)(w304, w302, w283, w256) -> (→"Graph 2":T12)
    n396 = Build Array (concatenate)(w298, w297, w281, w254) -> (→"Graph 4":T12)
    n397 = Build Array (concatenate)(w301, w299, w282, w255) -> (→"Graph 3":T12)
    "Cycle #" <- w260
  }
  n398 = call-dynamic "USBData_terminate.vi"("error in (no error)"=w19, "USBData in"=w20) -> ("error out"=w21:errorcluster)  [unwired: 8 in, 1 out]
  n399 = call-dynamic "LSI336Data_terminate.vi"("error in (no error)"=w8, "LSI336Data in"=w9) -> ("error out"=w7:errorcluster)  [unwired: 8 in, 1 out]
  n400 = call-dynamic "USBData_terminate.vi"("error in (no error)"=w1, "USBData in"=w2) -> ("error out"=w3:errorcluster)  [unwired: 8 in, 1 out]
  n401 = call "LSI218Data_terminate.vi"("error in (no error)"=w13, "LSI218Data in"=w14) -> ("error out"=w12:errorcluster)  [unwired: 8 in, 1 out]
  n402 = local write "error out (USB6210)"(w21) -> ()
  n403 = local write "error out (LSI336)"(w7) -> ()
  n404 = local write "error out (USB6210)"(w3) -> ()
  n405 = local write "error out (LSI218)"(w12) -> ()
